vi "SaccadeAnalyser - Main.vi"(8 "error in (no error)":errorcluster, 11 "Data IN":T3={"Impulse Positions"=[{"Start"=5471, "End"=5813, "Impulse Plane"=enum."Yaw", "Impulse Direction +ve?"=FALSE, "Time offset"=0, "Amplitude offset"=0.0}, {"Start"=6974, "End"=7325, "Impulse Plane"=enum."Yaw", "Impulse Direction +ve?"=TRUE, "Time offset"=0, "Amplitude offset"=0.0}, {"Start"=7641, "End"=7980, "Impulse Plane"=enum."Yaw", "Impulse Direction +ve?"=FALSE, "Time offset"=0, "Amplitude offset"=0.0}, {"Start"=9060, "End"=9400, "Impulse Plane"=enum."Yaw", "Impulse Direction +ve?"=FALSE, "Time offset"=0, "Amplitude offset"=0.0}, {"Start"=9938, "End"=10282, "Impulse Plane"=enum."Yaw", "Impulse Direction +ve?"=FALSE, "Time offset"=0, "Amplitude offset"=0.0}, {"Start"=10800, "End"=11142, "Impulse Plane"=enum."Yaw", "Impulse Direction +ve?"=FALSE, "Time offset"=0, "Amplitude offset"=0.0}, {"Start"=11602, "End"=11942, "Impulse Plane"=enum."Yaw", "Impulse Direction +ve?"=TRUE, "Time offset"=0, "Amplitude offset"=0.0}, {"Start"=12449, "End"=12790, "Impulse Plane"=enum."Yaw", "Impulse Direction +ve?"=TRUE, "Time offset"=0, "Amplitude offset"=0.0}, {"Start"=13310, "End"=13653, "Impulse Plane"=enum."Yaw", "Impulse Direction +ve?"=TRUE, "Time offset"=0, "Amplitude offset"=0.0}, {"Start"=14191, "End"=14535, "Impulse Plane"=enum."Yaw", "Impulse Direction +ve?"=TRUE, "Time offset"=0, "Amplitude offset"=0.0}, {"Start"=15040, "End"=15380, "Impulse Plane"=enum."Yaw", "Impulse Direction +ve?"=FALSE, "Time offset"=0, "Amplitude offset"=0.0}, {"Start"=16780, "End"=17124, "Impulse Plane"=enum."Yaw", "Impulse Direction +ve?"=TRUE, "Time offset"=0, "Amplitude offset"=0.0}, {"Start"=17572, "End"=17913, "Impulse Plane"=enum."Yaw", "Impulse Direction +ve?"=FALSE, "Time offset"=0, "Amplitude offset"=0.0}, {"Start"=18369, "End"=18713, "Impulse Plane"=enum."Yaw", "Impulse Direction +ve?"=FALSE, "Time offset"=0, "Amplitude offset"=0.0}, {"Start"=19174, "End"=19519, "Impulse Plane"=enum."Yaw", "Impulse Direction +ve?"=FALSE, "Time offset"=0, "Amplitude offset"=0.0}, {"Start"=19928, "End"=20270, "Impulse Plane"=enum."Yaw", "Impulse Direction +ve?"=TRUE, "Time offset"=0, "Amplitude offset"=0.0}, {"Start"=20762, "End"=21121, "Impulse Plane"=enum."Yaw", "Impulse Direction +ve?"=FALSE, "Time offset"=0, "Amplitude offset"=0.0}, {"Start"=21554, "End"=21888, "Impulse Plane"=enum."Yaw", "Impulse Direction +ve?"=FALSE, "Time offset"=0, "Amplitude offset"=0.0}, {"Start"=22293, "End"=22639, "Impulse Plane"=enum."Yaw", "Impulse Direction +ve?"=TRUE, "Time offset"=0, "Amplitude offset"=0.0}, {"Start"=23109, "End"=23464, "Impulse Plane"=enum."Yaw", "Impulse Direction +ve?"=TRUE, "Time offset"=0, "Amplitude offset"=0.0}, {"Start"=23868, "End"=24215, "Impulse Plane"=enum."Yaw", "Impulse Direction +ve?"=TRUE, "Time offset"=0, "Amplitude offset"=0.0}, {"Start"=24643, "End"=24992, "Impulse Plane"=enum."Yaw", "Impulse Direction +ve?"=FALSE, "Time offset"=0, "Amplitude offset"=0.0}, {"Start"=25685, "End"=26023, "Impulse Plane"=enum."Yaw", "Impulse Direction +ve?"=FALSE, "Time offset"=0, "Amplitude offset"=0.0}, {"Start"=26431, "End"=26768, "Impulse Plane"=enum."Yaw", "Impulse Direction +ve?"=FALSE, "Time offset"=0, "Amplitude offset"=0.0}, {"Start"=27251, "End"=27595, "Impulse Plane"=enum."Yaw", "Impulse Direction +ve?"=FALSE, "Time offset"=0, "Amplitude offset"=0.0}, {"Start"=28832, "End"=29180, "Impulse Plane"=enum."Yaw", "Impulse Direction +ve?"=TRUE, "Time offset"=0, "Amplitude offset"=0.0}, {"Start"=31028, "End"=31383, "Impulse Plane"=enum."LARP", "Impulse Direction +ve?"=FALSE, "Time offset"=0, "Amplitude offset"=0.0}, {"Start"=32603, "End"=32936, "Impulse Plane"=enum."LARP", "Impulse Direction +ve?"=TRUE, "Time offset"=0, "Amplitude offset"=0.0}, {"Start"=33445, "End"=33779, "Impulse Plane"=enum."LARP", "Impulse Direction +ve?"=TRUE, "Time offset"=0, "Amplitude offset"=0.0}, {"Start"=34276, "End"=34629, "Impulse Plane"=enum."LARP", "Impulse Direction +ve?"=FALSE, "Time offset"=0, "Amplitude offset"=0.0}, {"Start"=35114, "End"=35460, "Impulse Plane"=enum."LARP", "Impulse Direction +ve?"=FALSE, "Time offset"=0, "Amplitude offset"=0.0}, {"Start"=35981, "End"=36324, "Impulse Plane"=enum."LARP", "Impulse Direction +ve?"=TRUE, "Time offset"=0, "Amplitude offset"=0.0}, {"Start"=36920, "End"=37249, "Impulse Plane"=enum."LARP", "Impulse Direction +ve?"=TRUE, "Time offset"=0, "Amplitude offset"=0.0}, {"Start"=37988, "End"=38322, "Impulse Plane"=enum."LARP", "Impulse Direction +ve?"=TRUE, "Time offset"=0, "Amplitude offset"=0.0}, {"Start"=38964, "End"=39324, "Impulse Plane"=enum."LARP", "Impulse Direction +ve?"=FALSE, "Time offset"=0, "Amplitude offset"=0.0}, {"Start"=39948, "End"=40284, "Impulse Plane"=enum."LARP", "Impulse Direction +ve?"=TRUE, "Time offset"=0, "Amplitude offset"=0.0}, {"Start"=40958, "End"=41293, "Impulse Plane"=enum."LARP", "Impulse Direction +ve?"=TRUE, "Time offset"=0, "Amplitude offset"=0.0}, {"Start"=41899, "End"=42229, "Impulse Plane"=enum."LARP", "Impulse Direction +ve?"=TRUE, "Time offset"=0, "Amplitude offset"=0.0}, {"Start"=42801, "End"=43154, "Impulse Plane"=enum."LARP", "Impulse Direction +ve?"=FALSE, "Time offset"=0, "Amplitude offset"=0.0}, {"Start"=43641, "End"=43980, "Impulse Plane"=enum."LARP", "Impulse Direction +ve?"=TRUE, "Time offset"=0, "Amplitude offset"=0.0}, {"Start"=44466, "End"=44821, "Impulse Plane"=enum."LARP", "Impulse Direction +ve?"=FALSE, "Time offset"=0, "Amplitude offset"=0.0}, {"Start"=45388, "End"=45722, "Impulse Plane"=enum."LARP", "Impulse Direction +ve?"=TRUE, "Time offset"=0, "Amplitude offset"=0.0}, {"Start"=46149, "End"=46510, "Impulse Plane"=enum."LARP", "Impulse Direction +ve?"=FALSE, "Time offset"=0, "Amplitude offset"=0.0}, {"Start"=47874, "End"=48206, "Impulse Plane"=enum."LARP", "Impulse Direction +ve?"=TRUE, "Time offset"=0, "Amplitude offset"=0.0}, {"Start"=50143, "End"=50479, "Impulse Plane"=enum."RALP", "Impulse Direction +ve?"=TRUE, "Time offset"=0, "Amplitude offset"=0.0}, {"Start"=50976, "End"=51310, "Impulse Plane"=enum."RALP", "Impulse Direction +ve?"=FALSE, "Time offset"=0, "Amplitude offset"=0.0}, {"Start"=51892, "End"=52226, "Impulse Plane"=enum."RALP", "Impulse Direction +ve?"=FALSE, "Time offset"=0, "Amplitude offset"=0.0}, {"Start"=52839, "End"=53171, "Impulse Plane"=enum."RALP", "Impulse Direction +ve?"=FALSE, "Time offset"=0, "Amplitude offset"=0.0}, {"Start"=53676, "End"=54012, "Impulse Plane"=enum."RALP", "Impulse Direction +ve?"=TRUE, "Time offset"=0, "Amplitude offset"=0.0}, {"Start"=54530, "End"=54877, "Impulse Plane"=enum."RALP", "Impulse Direction +ve?"=FALSE, "Time offset"=0, "Amplitude offset"=0.0}, {"Start"=55371, "End"=55711, "Impulse Plane"=enum."RALP", "Impulse Direction +ve?"=TRUE, "Time offset"=0, "Amplitude offset"=0.0}, {"Start"=56153, "End"=56482, "Impulse Plane"=enum."RALP", "Impulse Direction +ve?"=FALSE, "Time offset"=0, "Amplitude offset"=0.0}, {"Start"=57053, "End"=57390, "Impulse Plane"=enum."RALP", "Impulse Direction +ve?"=FALSE, "Time offset"=0, "Amplitude offset"=0.0}, {"Start"=57954, "End"=58292, "Impulse Plane"=enum."RALP", "Impulse Direction +ve?"=FALSE, "Time offset"=0, "Amplitude offset"=0.0}, {"Start"=58794, "End"=59130, "Impulse Plane"=enum."RALP", "Impulse Direction +ve?"=TRUE, "Time offset"=0, "Amplitude offset"=0.0}, {"Start"=59587, "End"=59931, "Impulse Plane"=enum."RALP", "Impulse Direction +ve?"=TRUE, "Time offset"=0, "Amplitude offset"=0.0}, {"Start"=60399, "End"=60744, "Impulse Plane"=enum."RALP", "Impulse Direction +ve?"=FALSE, "Time offset"=0, "Amplitude offset"=0.0}, {"Start"=61218, "End"=61559, "Impulse Plane"=enum."RALP", "Impulse Direction +ve?"=FALSE, "Time offset"=0, "Amplitude offset"=0.0}, {"Start"=62100, "End"=62442, "Impulse Plane"=enum."RALP", "Impulse Direction +ve?"=FALSE, "Time offset"=0, "Amplitude offset"=0.0}, {"Start"=62989, "End"=63322, "Impulse Plane"=enum."RALP", "Impulse Direction +ve?"=FALSE, "Time offset"=0, "Amplitude offset"=0.0}, {"Start"=63787, "End"=64136, "Impulse Plane"=enum."RALP", "Impulse Direction +ve?"=TRUE, "Time offset"=0, "Amplitude offset"=0.0}, {"Start"=64603, "End"=64953, "Impulse Plane"=enum."RALP", "Impulse Direction +ve?"=FALSE, "Time offset"=0, "Amplitude offset"=0.0}, {"Start"=65462, "End"=65795, "Impulse Plane"=enum."RALP", "Impulse Direction +ve?"=FALSE, "Time offset"=0, "Amplitude offset"=0.0}, {"Start"=66308, "End"=66645, "Impulse Plane"=enum."RALP", "Impulse Direction +ve?"=FALSE, "Time offset"=0, "Amplitude offset"=0.0}, {"Start"=67052, "End"=67402, "Impulse Plane"=enum."RALP", "Impulse Direction +ve?"=TRUE, "Time offset"=0, "Amplitude offset"=0.0}], "No. Imp"=15, "Parameter Time Series"=[{"time offset"=0.0, "Offset"=0.0, "Gain"=1.0, "inverse"=FALSE, "filter data"=FALSE, "dots"=FALSE, "interpolate"=FALSE, "List 1"=5, "Color Box"=6618880, "Boolean"=TRUE}, {"time offset"=0.0, "Offset"=0.0, "Gain"=1.0, "inverse"=FALSE, "filter data"=FALSE, "dots"=FALSE, "interpolate"=FALSE, "List 1"=6, "Color Box"=6618880, "Boolean"=FALSE}, {"time offset"=0.0, "Offset"=0.0, "Gain"=1.0, "inverse"=FALSE, "filter data"=FALSE, "dots"=FALSE, "interpolate"=FALSE, "List 1"=7, "Color Box"=6618880, "Boolean"=FALSE}, {"time offset"=0.0, "Offset"=0.0, "Gain"=1.0, "inverse"=FALSE, "filter data"=FALSE, "dots"=FALSE, "interpolate"=FALSE, "List 1"=13, "Color Box"=16777224, "Boolean"=TRUE}, {"time offset"=0.0, "Offset"=0.0, "Gain"=1.0, "inverse"=FALSE, "filter data"=FALSE, "dots"=FALSE, "interpolate"=FALSE, "List 1"=14, "Color Box"=16777224, "Boolean"=FALSE}, {"time offset"=0.0, "Offset"=0.0, "Gain"=1.0, "inverse"=FALSE, "filter data"=FALSE, "dots"=FALSE, "interpolate"=FALSE, "List 1"=15, "Color Box"=16777224, "Boolean"=FALSE}], "Parameter Impuls Series"=[{"Color"=6618880, "Visible"=TRUE, "Channel"=1, "Invert"=FALSE, "Desaccade"=FALSE, "Offset"=0.0, "Gain"=1.0}, {"Color"=6618880, "Visible"=FALSE, "Channel"=6, "Invert"=FALSE, "Desaccade"=FALSE, "Offset"=0.0, "Gain"=1.0}, {"Color"=6618880, "Visible"=FALSE, "Channel"=7, "Invert"=FALSE, "Desaccade"=FALSE, "Offset"=0.0, "Gain"=1.0}, {"Color"=16777224, "Visible"=TRUE, "Channel"=13, "Invert"=FALSE, "Desaccade"=FALSE, "Offset"=0.0, "Gain"=1.0}, {"Color"=16777224, "Visible"=FALSE, "Channel"=14, "Invert"=FALSE, "Desaccade"=FALSE, "Offset"=0.0, "Gain"=1.0}, {"Color"=16777224, "Visible"=FALSE, "Channel"=15, "Invert"=FALSE, "Desaccade"=FALSE, "Offset"=0.0, "Gain"=1.0}], "Experiment Parameters"={"Freq"=0.0, "Vel"=0, "Acc"=0, "Stimulus"="Head Impulse"}, "Autosort File"=refnum, "Data File"={"Data Channels"=array34x71049[2415666 elements], "Sample Rate"=500, "Channel List"=["Hz Position-in-Head", "Hz Velocity-in-Head", "Hy Position-in-Head", "Hy Velocity-in-Head", "Hx Position-in-Head", "Hx Velocity-in-Head", "Hl Velocity-in-Head", "Hr Velocity-in-Head", "Lx Position-in-Head", "Ly Position-in-Head", "Lz Position-in-Head", "Lx Velocity-in-Head", "Ly Velocity-in-Head", "Lz Velocity-in-Head", "Ll Velocity-in-Head", "Lr Velocity-in-Head", "Rx Position-in-Head", "Ry Position-in-Head", "Rz Position-in-Head", "Rx Velocity-in-Head", "Ry Velocity-in-Head", "Rz Velocity-in-Head", "Rl Velocity-in-Head", "Rr Velocity-in-Head", "Target on/off", "aux input 1", "aux input 2", " ", "", "", "", "Target Hor", "Target Ver", ""]}, "Experiment data path"=path "C:/Users/w.figtree/Desktop/Coils Data/3", "Image data path"=path "/Macintosh HD/Users/patrick/Studium/Diploma Thesis/Data Analysis", "LVS data path"=path "/Macintosh HD/Users/patrick/Studium/Diploma Thesis/Data Analysis", "Raw copy path"=path "/Macintosh HD/Users/patrick/Studium/Diploma Thesis/Data Analysis", "filename"="passive_lvs.lvs", "desaccading parameters"={"Tolerance"=3, "Acc Range"=7000.0, "Sample Rate"=500, "Impulse Plane 2"=enum."Yaw", "Impulse dir"=FALSE}, "Experiment Parameters 2"={"Subject"="SE Trial Short Term", "Strain"="", "Rotation plane"="", "Experimenter"=" ", "Trial"=0.0, "Time"=0.0}, "Excel"={"Excel._Application"=refnum, "Use Excel"=TRUE, "Worksheet SINE"=refnum, "Row SINE"=0, "Worksheet TRANS"=refnum, "Row TRANS"=0}, "Session Config File"=refnum, "Autosort Parameter Set"=4, "EMA Version"="EMA 2016a", "desacc "={"Threshold 1 [Acc]"=7000.0, "Threshold 2 [% of TH1]"=60, "tolerance"=3, "Search WD "=0.1, " always use TH2"=FALSE, "Range"=3.0, "Max time"=120.0, "Min time"=20.0, "Velocity Threshold"=150}, "Cycle Nr for Saccades"={"POS"=0, "NEG"=0}, "calibration name"="u_calibration_1_p00001s001_calib.mat", "Excel"=refnum} {"Parameter Time Series"."time offset" format="%.3f"; "Parameter Time Series"."Gain" format="%.1f"; "Parameter Time Series"."Offset" format="%.1f"; "Parameter Time Series"."List 1" items=["Motor-Pos", "Motor-Vel", "Lx Position-in-Head", "Ly Position-in-Head", "Lz Position-in-Head", "Lx Velocity-in-Head", "Ly Velocity-in-Head", "Lz Velocity-in-Head", "Ll Velocity-in-Head", "Lr Velocity-in-Head", "Lx Accel-in-Head", "Ly Accel-in-Head", "Lz Accel-in-Head", "Rx Position-in-Head", "Ry Position-in-Head", "Rz Position-in-Head", "Rx Velocity-in-Head", "Ry Velocity-in-Head", "Rz Velocity-in-Head", "Rl Velocity-in-Head", "Rr Velocity-in-Head", "Rx Accel-in-Head", "Ry Accel-in-Head", "Rz Accel-in-Head", "Global Trigger", "", "", ""]; "Parameter Impuls Series"."Gain" format="%.1f"; "Parameter Impuls Series"."Offset" format="%.1f"}) -> (0 "error out":errorcluster, 3 "Data OUT":T3={"Impulse Positions"=[{"Start"=5471, "End"=5813, "Impulse Plane"=enum."Yaw", "Impulse Direction +ve?"=FALSE, "Time offset"=0, "Amplitude offset"=0.0}, {"Start"=6974, "End"=7325, "Impulse Plane"=enum."Yaw", "Impulse Direction +ve?"=TRUE, "Time offset"=0, "Amplitude offset"=0.0}, {"Start"=7641, "End"=7980, "Impulse Plane"=enum."Yaw", "Impulse Direction +ve?"=FALSE, "Time offset"=0, "Amplitude offset"=0.0}, {"Start"=9060, "End"=9400, "Impulse Plane"=enum."Yaw", "Impulse Direction +ve?"=FALSE, "Time offset"=0, "Amplitude offset"=0.0}, {"Start"=9938, "End"=10282, "Impulse Plane"=enum."Yaw", "Impulse Direction +ve?"=FALSE, "Time offset"=0, "Amplitude offset"=0.0}, {"Start"=10800, "End"=11142, "Impulse Plane"=enum."Yaw", "Impulse Direction +ve?"=FALSE, "Time offset"=0, "Amplitude offset"=0.0}, {"Start"=11602, "End"=11942, "Impulse Plane"=enum."Yaw", "Impulse Direction +ve?"=TRUE, "Time offset"=0, "Amplitude offset"=0.0}, {"Start"=12449, "End"=12790, "Impulse Plane"=enum."Yaw", "Impulse Direction +ve?"=TRUE, "Time offset"=0, "Amplitude offset"=0.0}, {"Start"=13310, "End"=13653, "Impulse Plane"=enum."Yaw", "Impulse Direction +ve?"=TRUE, "Time offset"=0, "Amplitude offset"=0.0}, {"Start"=14191, "End"=14535, "Impulse Plane"=enum."Yaw", "Impulse Direction +ve?"=TRUE, "Time offset"=0, "Amplitude offset"=0.0}, {"Start"=15040, "End"=15380, "Impulse Plane"=enum."Yaw", "Impulse Direction +ve?"=FALSE, "Time offset"=0, "Amplitude offset"=0.0}, {"Start"=16780, "End"=17124, "Impulse Plane"=enum."Yaw", "Impulse Direction +ve?"=TRUE, "Time offset"=0, "Amplitude offset"=0.0}, {"Start"=17572, "End"=17913, "Impulse Plane"=enum."Yaw", "Impulse Direction +ve?"=FALSE, "Time offset"=0, "Amplitude offset"=0.0}, {"Start"=18369, "End"=18713, "Impulse Plane"=enum."Yaw", "Impulse Direction +ve?"=FALSE, "Time offset"=0, "Amplitude offset"=0.0}, {"Start"=19174, "End"=19519, "Impulse Plane"=enum."Yaw", "Impulse Direction +ve?"=FALSE, "Time offset"=0, "Amplitude offset"=0.0}, {"Start"=19928, "End"=20270, "Impulse Plane"=enum."Yaw", "Impulse Direction +ve?"=TRUE, "Time offset"=0, "Amplitude offset"=0.0}, {"Start"=20762, "End"=21121, "Impulse Plane"=enum."Yaw", "Impulse Direction +ve?"=FALSE, "Time offset"=0, "Amplitude offset"=0.0}, {"Start"=21554, "End"=21888, "Impulse Plane"=enum."Yaw", "Impulse Direction +ve?"=FALSE, "Time offset"=0, "Amplitude offset"=0.0}, {"Start"=22293, "End"=22639, "Impulse Plane"=enum."Yaw", "Impulse Direction +ve?"=TRUE, "Time offset"=0, "Amplitude offset"=0.0}, {"Start"=23109, "End"=23464, "Impulse Plane"=enum."Yaw", "Impulse Direction +ve?"=TRUE, "Time offset"=0, "Amplitude offset"=0.0}, {"Start"=23868, "End"=24215, "Impulse Plane"=enum."Yaw", "Impulse Direction +ve?"=TRUE, "Time offset"=0, "Amplitude offset"=0.0}, {"Start"=24643, "End"=24992, "Impulse Plane"=enum."Yaw", "Impulse Direction +ve?"=FALSE, "Time offset"=0, "Amplitude offset"=0.0}, {"Start"=25685, "End"=26023, "Impulse Plane"=enum."Yaw", "Impulse Direction +ve?"=FALSE, "Time offset"=0, "Amplitude offset"=0.0}, {"Start"=26431, "End"=26768, "Impulse Plane"=enum."Yaw", "Impulse Direction +ve?"=FALSE, "Time offset"=0, "Amplitude offset"=0.0}, {"Start"=27251, "End"=27595, "Impulse Plane"=enum."Yaw", "Impulse Direction +ve?"=FALSE, "Time offset"=0, "Amplitude offset"=0.0}, {"Start"=28832, "End"=29180, "Impulse Plane"=enum."Yaw", "Impulse Direction +ve?"=TRUE, "Time offset"=0, "Amplitude offset"=0.0}, {"Start"=31028, "End"=31383, "Impulse Plane"=enum."LARP", "Impulse Direction +ve?"=FALSE, "Time offset"=0, "Amplitude offset"=0.0}, {"Start"=32603, "End"=32936, "Impulse Plane"=enum."LARP", "Impulse Direction +ve?"=TRUE, "Time offset"=0, "Amplitude offset"=0.0}, {"Start"=33445, "End"=33779, "Impulse Plane"=enum."LARP", "Impulse Direction +ve?"=TRUE, "Time offset"=0, "Amplitude offset"=0.0}, {"Start"=34276, "End"=34629, "Impulse Plane"=enum."LARP", "Impulse Direction +ve?"=FALSE, "Time offset"=0, "Amplitude offset"=0.0}, {"Start"=35114, "End"=35460, "Impulse Plane"=enum."LARP", "Impulse Direction +ve?"=FALSE, "Time offset"=0, "Amplitude offset"=0.0}, {"Start"=35981, "End"=36324, "Impulse Plane"=enum."LARP", "Impulse Direction +ve?"=TRUE, "Time offset"=0, "Amplitude offset"=0.0}, {"Start"=36920, "End"=37249, "Impulse Plane"=enum."LARP", "Impulse Direction +ve?"=TRUE, "Time offset"=0, "Amplitude offset"=0.0}, {"Start"=37988, "End"=38322, "Impulse Plane"=enum."LARP", "Impulse Direction +ve?"=TRUE, "Time offset"=0, "Amplitude offset"=0.0}, {"Start"=38964, "End"=39324, "Impulse Plane"=enum."LARP", "Impulse Direction +ve?"=FALSE, "Time offset"=0, "Amplitude offset"=0.0}, {"Start"=39948, "End"=40284, "Impulse Plane"=enum."LARP", "Impulse Direction +ve?"=TRUE, "Time offset"=0, "Amplitude offset"=0.0}, {"Start"=40958, "End"=41293, "Impulse Plane"=enum."LARP", "Impulse Direction +ve?"=TRUE, "Time offset"=0, "Amplitude offset"=0.0}, {"Start"=41899, "End"=42229, "Impulse Plane"=enum."LARP", "Impulse Direction +ve?"=TRUE, "Time offset"=0, "Amplitude offset"=0.0}, {"Start"=42801, "End"=43154, "Impulse Plane"=enum."LARP", "Impulse Direction +ve?"=FALSE, "Time offset"=0, "Amplitude offset"=0.0}, {"Start"=43641, "End"=43980, "Impulse Plane"=enum."LARP", "Impulse Direction +ve?"=TRUE, "Time offset"=0, "Amplitude offset"=0.0}, {"Start"=44466, "End"=44821, "Impulse Plane"=enum."LARP", "Impulse Direction +ve?"=FALSE, "Time offset"=0, "Amplitude offset"=0.0}, {"Start"=45388, "End"=45722, "Impulse Plane"=enum."LARP", "Impulse Direction +ve?"=TRUE, "Time offset"=0, "Amplitude offset"=0.0}, {"Start"=46149, "End"=46510, "Impulse Plane"=enum."LARP", "Impulse Direction +ve?"=FALSE, "Time offset"=0, "Amplitude offset"=0.0}, {"Start"=47874, "End"=48206, "Impulse Plane"=enum."LARP", "Impulse Direction +ve?"=TRUE, "Time offset"=0, "Amplitude offset"=0.0}, {"Start"=50143, "End"=50479, "Impulse Plane"=enum."RALP", "Impulse Direction +ve?"=TRUE, "Time offset"=0, "Amplitude offset"=0.0}, {"Start"=50976, "End"=51310, "Impulse Plane"=enum."RALP", "Impulse Direction +ve?"=FALSE, "Time offset"=0, "Amplitude offset"=0.0}, {"Start"=51892, "End"=52226, "Impulse Plane"=enum."RALP", "Impulse Direction +ve?"=FALSE, "Time offset"=0, "Amplitude offset"=0.0}, {"Start"=52839, "End"=53171, "Impulse Plane"=enum."RALP", "Impulse Direction +ve?"=FALSE, "Time offset"=0, "Amplitude offset"=0.0}, {"Start"=53676, "End"=54012, "Impulse Plane"=enum."RALP", "Impulse Direction +ve?"=TRUE, "Time offset"=0, "Amplitude offset"=0.0}, {"Start"=54530, "End"=54877, "Impulse Plane"=enum."RALP", "Impulse Direction +ve?"=FALSE, "Time offset"=0, "Amplitude offset"=0.0}, {"Start"=55371, "End"=55711, "Impulse Plane"=enum."RALP", "Impulse Direction +ve?"=TRUE, "Time offset"=0, "Amplitude offset"=0.0}, {"Start" (continued)
      }
      frame "Enable Controls" {
        # "Enable everything"
        # "Enable all front panel controls, allowing user interaction."
        n372 = call <userlib>:"MGI Get VI Control Ref[].vi"() -> ("error out"=w681:errorcluster, "Control[i]"=w682:refnum<vi>[])  [unwired: 8 in, 2 out]
        n373 = call <vilib>:"Enable Group.vi"("error in (no error)"=w681, "Group"=w682) -> ("error out"=w679:errorcluster)  [unwired: 8 in, 1 out]
        n374 = property on="mclb_summary" class="MCListbox (strict)"(error in=w679, "DisabledEnum"=T18."Disabled" ("Disabled")) -> ()  [unwired: 1 in, 2 out]
      }
      frame "Give MCLB Focus" {
        # "Gives key focus to the Saccade MCLB. Required after some operations (e.g. Draw)."
        n375 = property on="mclb_saccades" class="MCListbox (strict)"("Key Focus"=TRUE) -> ()  [unwired: 2 in, 2 out]
      }
      frame "Toggle Saccade" {
        # "Toggle the inclusion status of the currently selected saccade."
        n376 = local read "mclb_saccades"() -> (w693:i32)
        n377 = Unbundle By Name(w692) -> ("Saccades"=w694:T8[])
        n378 = in-place {
          n379 = in-place-array #6(w694, w693) -> (w699:T8)
          n380 = Unbundle By Name(w699) -> ("Included?"=w698:bool)
          n381 = Not(x=w698) -> (.not. x?=w697:bool)
          n382 = Bundle By Name(cluster=w699, "Included?"=w697) -> (w700:T8)
          n383 = in-place-array #6(w700) -> (w690:T8[])  [unwired: 1 out]
        }
        n384 = Bundle By Name(cluster=w692, "Saccades"=w690) -> (w691:T6)
      }
      frame "DO - Export Summary" {
        w701 = T10[] [enum."Export - Open Summary", enum."Export - Summary", enum."Give MCLB Focus"] items=["Initialise", "Quit", "DO - Analysis", "DO - Summary Analysis", "Load Channel Data", "Find Impulses", "Find Saccades", "Sequence Saccades", "Calc Saccade Summary Stats", "Calc Saccade Group Stats", "DO - Draw", "Clear Plot", "Plot Selected Saccade", "Plot Selected Saccade Siblings", "Plot Impulse Data", "Plot Saccade Data", "Fill Saccade MCLB", "Fill Summary Stats", "Give MCLB Focus", "Halt Panel Updates", "Resume Panel Updates", "Disable Controls", "Enable Controls", "Toggle Saccade", "DO - Export Summary", "Export - Open Summary", "Export - Summary", "DO - Export Saccades", "Export - Open Saccades", "Export - Saccades", "DO - Export Group", "Export - Open Group", "Export - Group", "Do - Export All"] ("element")
        # "Enqueue export summary process states."
        n385 = for {
          tunnel: w702 -> [w707]
          tunnel: w701 -> [w706] mode=indexing
          n386 = Enqueue Element(queue=w707, element=w706) -> ()  [unwired: 2 in, 3 out]
        }
      }
      frame "DO - Export Group" {
        w708 = T10[] [enum."Export - Open Group", enum."Export - Group", enum."Give MCLB Focus"] items=["Initialise", "Quit", "DO - Analysis", "DO - Summary Analysis", "Load Channel Data", "Find Impulses", "Find Saccades", "Sequence Saccades", "Calc Saccade Summary Stats", "Calc Saccade Group Stats", "DO - Draw", "Clear Plot", "Plot Selected Saccade", "Plot Selected Saccade Siblings", "Plot Impulse Data", "Plot Saccade Data", "Fill Saccade MCLB", "Fill Summary Stats", "Give MCLB Focus", "Halt Panel Updates", "Resume Panel Updates", "Disable Controls", "Enable Controls", "Toggle Saccade", "DO - Export Summary", "Export - Open Summary", "Export - Summary", "DO - Export Saccades", "Export - Open Saccades", "Export - Saccades", "DO - Export Group", "Export - Open Group", "Export - Group", "Do - Export All"] ("element")
        # "Enqueue export group process states."
        n387 = for {
          tunnel: w709 -> [w714]
          tunnel: w708 -> [w713] mode=indexing
          n388 = Enqueue Element(queue=w714, element=w713) -> ()  [unwired: 2 in, 3 out]
        }
      }
      frame "DO - Export Saccades" {
        w716 = T10[] [enum."Export - Open Saccades", enum."Export - Saccades", enum."Give MCLB Focus"] items=["Initialise", "Quit", "DO - Analysis", "DO - Summary Analysis", "Load Channel Data", "Find Impulses", "Find Saccades", "Sequence Saccades", "Calc Saccade Summary Stats", "Calc Saccade Group Stats", "DO - Draw", "Clear Plot", "Plot Selected Saccade", "Plot Selected Saccade Siblings", "Plot Impulse Data", "Plot Saccade Data", "Fill Saccade MCLB", "Fill Summary Stats", "Give MCLB Focus", "Halt Panel Updates", "Resume Panel Updates", "Disable Controls", "Enable Controls", "Toggle Saccade", "DO - Export Summary", "Export - Open Summary", "Export - Summary", "DO - Export Saccades", "Export - Open Saccades", "Export - Saccades", "DO - Export Group", "Export - Open Group", "Export - Group", "Do - Export All"] ("element")
        # "Enqueue export all saccades process states."
        n389 = for {
          tunnel: w715 -> [w721]
          tunnel: w716 -> [w720] mode=indexing
          n390 = Enqueue Element(queue=w721, element=w720) -> ()  [unwired: 2 in, 3 out]
        }
      }
      frame "Export - Open Summary" {
        # "Use provided sheet name or fall back to a default"
        # "Opens an Excel instance, workbook, and summary worksheet."
        n391 = local read "export_SaccadesSheet"() -> (w731:string)
        n392 = Empty String/Path?(string/path=w731) -> (empty?=w732:bool)
        n393 = Select(t="Saccades", s=w732, f=w731) -> (s? t:f=w727:string)
        n394 = Unbundle By Name(w724) -> ("Excel"=w729:refnum<class "Excel.lvclass">)
        n395 = Concatenate Strings(w727, " Summary" ("string")) -> (w726:string)
        n396 = call <userlib>:"Open.vi"("Worksheet Name (Sheet1)"=w726, "Excel in"=w729) -> ("Excel out"=w728:refnum<class "Excel.lvclass">)  [unwired: 8 in, 1 out]
        n397 = Bundle By Name(cluster=w724, "Excel"=w728) -> (w723:T3)
      }
      frame "Export - Summary" {
        # "Save the workbook."
        # "Write data"
        # "Write header"
        # "Exports summary data to an open Excel sheet."
        n398 = property on="enum_plane" class="Enum (strict)"() -> ("Strings []"=w765:string[], "Value"=w764:T14)  [unwired: 2 in, 2 out]
        n399 = property on="enum_direction" class="Enum (strict)"() -> ("Strings []"=w762:string[], "Value"=w763:enum16{"Positive", "Negative"})  [unwired: 2 in, 2 out]
        n400 = property on="enum_summaryType" class="Enum (strict)"() -> ("Strings []"=w761:string[], "Value"=w760:enum16{"Mean", "Median"})  [unwired: 2 in, 2 out]
        n401 = Unbundle By Name(w735) -> ("Summary"=w747:T9)
        n402 = Unbundle By Name(w735) -> ("Num Impulses"=w734:i32)
        n403 = Unbundle By Name(w745) -> ("Experiment Parameters 2.Subject"=w759:string)
        n404 = Unbundle By Name(w745) -> ("Excel"=w746:refnum<class "Excel.lvclass">)
        n405 = Index Array(array=w765, index=w764) -> (element=w758:string)
        n406 = Index Array(array=w762, index=w763) -> (element=w757:string)
        n407 = Index Array(array=w761, index=w760) -> (element=w756:string)
        n408 = Unbundle By Name(w747) -> ("Num Impulses"=w749:dbl, "Num Saccades"=w748:dbl, "Onset (ms)"=w754:dbl, "Duration (ms)"=w753:dbl, "Vel (°/s)"=w751:dbl, "Amplitude (°)"=w750:dbl, "Gain"=w752:dbl)
        n409 = Build Array(w734, w749, w748) -> (w740:dbl[])
        n410 = Build Array(w759, w758, w757, w756) -> (w741:string[])
        n411 = Build Array(w754, w753, w751, w750, w752) -> (w739:dbl[])
        n412 = Number To Decimal String(number=w740) -> (decimal integer string=w738:string[])  [unwired: 1 in]
        n413 = Number To Fractional String(number=w739) -> (F-format string=w737:string[])  [unwired: 3 in]
        n414 = Build Array (concatenate)(w741, w738, w737) -> (w736:string[])
        n415 = call <userlib>:"Write.vi"("Cell (Append to next row)"=cluster{"Row":i32, "Col":i32} {"Row"=0, "Col"=0}, "Data"=string[] ["Subject", "Plane", "Direction", "Summary Method", "Total Impulses", "Number of Impulses", "Number of Saccades", "Onset (ms)", "Duration (ms)", "Velocity (°/s)", "Amplitude (°)", "Gain"], "Excel in"=w746) -> ("error out"=w767:errorcluster, "Excel out"=w768:refnum<class "Excel.lvclass">)  [unwired: 6 in, 1 out]
        n416 = call <userlib>:"Write.vi"("error in (no error)"=w767, "Data"=w736, "Excel in"=w768) -> ("error out"=w742:errorcluster, "Excel out"=w743:refnum<class "Excel.lvclass">)  [unwired: 6 in, 1 out]
        n417 = call <userlib>:"Save.vi"("error in (no error)"=w742, "Excel in"=w743) -> ("Excel out"=w766:refnum<class "Excel.lvclass">)  [unwired: 7 in, 2 out]
        n418 = Bundle By Name(cluster=w745, "Excel"=w766) -> (w744:T3)
      }
      frame "Export - Open Group" {
        # "Use provided sheet name or fall back to a default"
        # "Opens an Excel instance, workbook, and summary worksheet."
        n419 = local read "export_SaccadesSheet"() -> (w780:string)
        n420 = Empty String/Path?(string/path=w780) -> (empty?=w781:bool)
        n421 = Select(t="Saccades", s=w781, f=w780) -> (s? t:f=w776:string)
        n422 = Unbundle By Name(w773) -> ("Excel"=w778:refnum<class "Excel.lvclass">)
        n423 = Concatenate Strings(w776, " Group Summary" ("string")) -> (w775:string)
        n424 = call <userlib>:"Open.vi"("Worksheet Name (Sheet1)"=w775, "Excel in"=w778) -> ("Excel out"=w777:refnum<class "Excel.lvclass">)  [unwired: 8 in, 1 out]
        n425 = Bundle By Name(cluster=w773, "Excel"=w777) -> (w772:T3)
      }
      frame "Export - Group" {
        # "Build Numeric portion of the header"
        # "Build constant string data"
        # "Add on constant header portion"
        # "Save the workbook."
        # "Write data"
        # "Write header"
        # "Exports group summary data to an open Excel sheet."
        n426 = Unbundle By Name(w791) -> ("Group Summary"=w792:T9[])
        n427 = for {
          tunnel: [w824] -> w794 mode=concatenating
          tunnel: w792 -> [w819] mode=indexing
          tunnel: [w811] -> w785 mode=concatenating
          i -> [w822]
          # "Build numeric data"
          n428 = Cluster To Array(cluster=w819) -> (array=w816:dbl[])
          n429 = Delete From Array(array=w816, length=2, index=0) -> (deleted portion=w815:dbl[], array with subset deleted=w814:dbl[])
          n430 = Format Into String(format string="S%d_", w822) -> (resulting string=w821:string)  [unwired: 2 in, 1 out]
          n431 = Number To Decimal String(number=w815) -> (decimal integer string=w812:string[])  [unwired: 1 in]
          n432 = Number To Fractional String(number=w814) -> (F-format string=w813:string[])  [unwired: 3 in]
          n433 = for {
            tunnel: w821 -> [w827]
            tunnel: string[] ["Number of Impulses", "Number of Saccades", "Onset (ms)", "Onset SD (ms)", "Duration (ms)", "Duration SD (ms)", "Velocity (°/s)", "Velocity SD (°/s)", "Amplitude (°)", "Amplitude SD (°)", "Gain", "Gain SD"] -> [w826] mode=indexing
            tunnel: [w825] -> w824 mode=indexing
            n434 = Concatenate Strings(w827, w826) -> (w825:string)
          }
          n435 = Build Array (concatenate)(w812, w813) -> (w811:string[])
        }
        n436 = Build Array (concatenate)(string[] ["Subject", "Plane", "Direction", "Summary Method"], w794) -> (w793:string[])
        n437 = Unbundle By Name(w789) -> ("Excel"=w788:refnum<class "Excel.lvclass">)
        n438 = property on="enum_plane" class="Enum (strict)"() -> ("Strings []"=w805:string[], "Value"=w804:T14)  [unwired: 2 in, 2 out]
        n439 = property on="enum_direction" class="Enum (strict)"() -> ("Strings []"=w802:string[], "Value"=w803:enum16{"Positive", "Negative"})  [unwired: 2 in, 2 out]
        n440 = property on="enum_summaryType" class="Enum (strict)"() -> ("Strings []"=w801:string[], "Value"=w800:enum16{"Mean", "Median"})  [unwired: 2 in, 2 out]
        n441 = Unbundle By Name(w789) -> ("Experiment Parameters 2.Subject"=w799:string)
        n442 = Index Array(array=w805, index=w804) -> (element=w798:string)